vi "Modelo planta H2_V3.vi"() -> ()   [LabVIEW 2024]
uses:
  <vilib>/Modbus/master/Create Master Instance (TCP).vi
  <vilib>/Modbus/master/Modbus Master.lvclass
  <vilib>/OPCUA/NI OPC UA Client.lvlib
  SALICRU_MODBUS.lvlib
  S7-1200_OPCUA.lvlib
panel:
  out "EV6":bool caption="Not initialized"
  out "EV5":bool caption="Not initialized"
  out "EV4":bool caption="Not initialized"
  out "EV3":bool caption="Idle"
  out "EV2":bool caption="Not initialized"
  out "EV1":bool caption="Stand By"
  out "x-y 4":u32
  out "x-y 3":u32
  in  "Restart INV SALICRU com":bool
  in  "Restart SAI com":bool
  out "x-y 2":u32
  in  "stop":bool
  out "x-y":u32
  in  "Tab Control":enum32{"Vista General", "Producción", "Energía"}(tab)
  out "E2.14 2":bool caption="Not initialized"
  out "E1.1":bool caption="Maintenance mode"
  out "E2.2":bool caption="Not initialized"
  out "E2.3":bool caption="Not initialized"
  out "E1.2":bool caption="Maintenance mode"
  out "E1.3":bool caption="Idle"
  out "Prod electrolizadores (display) 4":dbl format="%#.4g"
  out "Prod electrolizadores (display) 3":dbl format="%#.4g"
  out "Prod electrolizadores (display) 2":dbl format="%#.4g"
  out "Potenica Solar (Display) 2":dbl format="%#.2f"
  out "masa total G Kg 2":dbl format="%#.3f"
  out "P alta 2":dbl format="%.1f"
  out "P baja 2":dbl format="%.1f"
  out "masa total P Kg  2":dbl format="%#.3f"
  in  "SAI":bool caption="Line"
  out "Potenica Solar (Display) 3":dbl format="%#.2f"
  out "Comunicacion SAI":bool
  out "E2.1":bool caption="Not initialized"
  out "E2.2":bool caption="Not initialized"
  out "E1.2 2":bool caption="Idle"
  out "E1.1,2":bool caption="Maintenance mode"
  out "E2.1 3":bool caption="Not initialized"
  out "E1.2":bool caption="Maintenance mode"
  out "Producció d'hidrogen":dbl(graph)
  out "Energia solar no utilitzada":dbl(graph)
  out "Pressió tanc baixa":dynamicdata(graph)
  out "Potenica Solar (Display)":dbl format="%#.2f"
  out "Producción FC":dbl format="%#_2g"
  out "Prod electrolizadores (display)":dbl format="%#.4g"
  out "P baja":dbl format="%.1f"
  out "masa total G Kg":dbl format="%#.0f"
  out "Potència inversor solar":dynamicdata(graph)
  out "Watimetro ARPA":dbl format="%#.1f"
  out "masa total P Kg":dbl format="%#.1f"
  out "Compresor":bool
  out "P alta":dbl format="%.1f"
  out "Tèrmic\nExtractors":bool
  out "Relé Seguretat":bool
  out "Sobretensions":bool
  out "Baliza verde":bool
  out "Baliza amarilla":bool
  out "Baliza roja":bool
  out "H2 generado Total":dbl format="%#.1f"
  out "Producción Solar toral":dbl format="%#.1f"
  out "Energía acum H2 verde":dbl format="%#.1f"
  out "H2 consumido en el lab":dbl=182.6 format="%#.1f"
  out "Energía solar diaría":dbl format="%#.1f"
  out "H2 generado dia":dbl format="%#.1f"
  out "Comunicacion Inversor SALICRU":bool
  out "Tank":dbl(slide) scale=0.0..10.0
  out "P tanq alta (barg)":dbl(graph)
  in  "Energía acum H2 verde inicio":dbl=527.0
  in  "Producción Solar total inicio":dbl=3421.0
  in  "H2 generado inicio":dbl=202.8
  out "g H2 consumidos por la FC":dbl
  out "g comprimidos":dbl
  in  "Caudal compresor":dbl
  out "P tanq baja (barg)":dbl(graph)
  in  "Presión ini Tanq baba":dbl=28.0
  in  "Presión ini Tanq alta":dbl=220.0
  out "Energía Solar no usada (kWh)":dbl(graph)
  out "H2 acumulado diario (g)":dbl(graph)
  out "Producción instalan (g/s)":dbl(graph)
  out "Electroli ON":dbl(graph)
  out "Potencia Consumo electroli instan. (kW)":dbl(graph)
  out "Producción diaria (g)":dbl
  out "Producción instalan (g/s)":dbl
  out "Electroli ON":dbl
  out "Potencia Solar Instanta (kW)":dbl(graph)
  # "EV1"
  # "EV4"
  # "ESTADO ELECTROVÁLVULAS"
  # "EV5"
  # "EV2"
  # "EV3"
  # "EV6"
  # "g"
  # "bar"
  # "bar"
  # "kg"
  # "kWh"
  # "kWh"
  # "Ambiente"
  # "Temperatura"
  # "ºC"
  # "Humedad"
  # "%"
  # "ESTADO ELY"
  # "E1.1"
  # "E2.1"
  # "E1.2"
  # "E2.2"
  # "E2.3"
  # "E1.3"
  # "Modo:"
  # "RESUMEN DE LA PRODUCCIÓN"
  # "SAI PLANTA"
  # "Electrolizadores"
  # "Producción\nElectrolizadores:"
  # "g/s"
  # "Inversor solar:"
  # "Energía solar:"
  # "kW"
  # "Tanque Alta"
  # "Presión:"
  # "barg"
  # "Kg"
  # "Capacidad:"
  # "Tanque Baja"
  # "Presión:"
  # "barg"
  # "Kg"
  # "Capacidad:"
  # "SAI:"
  # "Potencia (%):"
  # "%"
  # "Seguretat"
  # "H2 baixa pressió"
  # "H2 alta pressió"
  # "barg"
  # "Tanc baixa pressió"
  # "Tanc alta pressió"
  # "Compressor"
  # "barg"
  # "Solar"
  # "Fuel Cell"
  # "kW"
  # "kW"
  # "Kg"
  # "Kg"
  # "Electrolizadores"
  # "g/s"
  # "Xarxa electrica"
  # "-"
  # "+"
  # "kW de xarxa"
  # "Producció total d'hidrogen"
  # "Producció d'hidrogen diària"
  # "g"
  # "kg"
  # "Producció total d'energia solar"
  # "Energia solar produïda diària"
  # "kWh"
  # "kWh"
  # "Energia acumulada per H2 verd"
  # "Consum de H2 Lab diari"
  # "g"
  # "kWh"
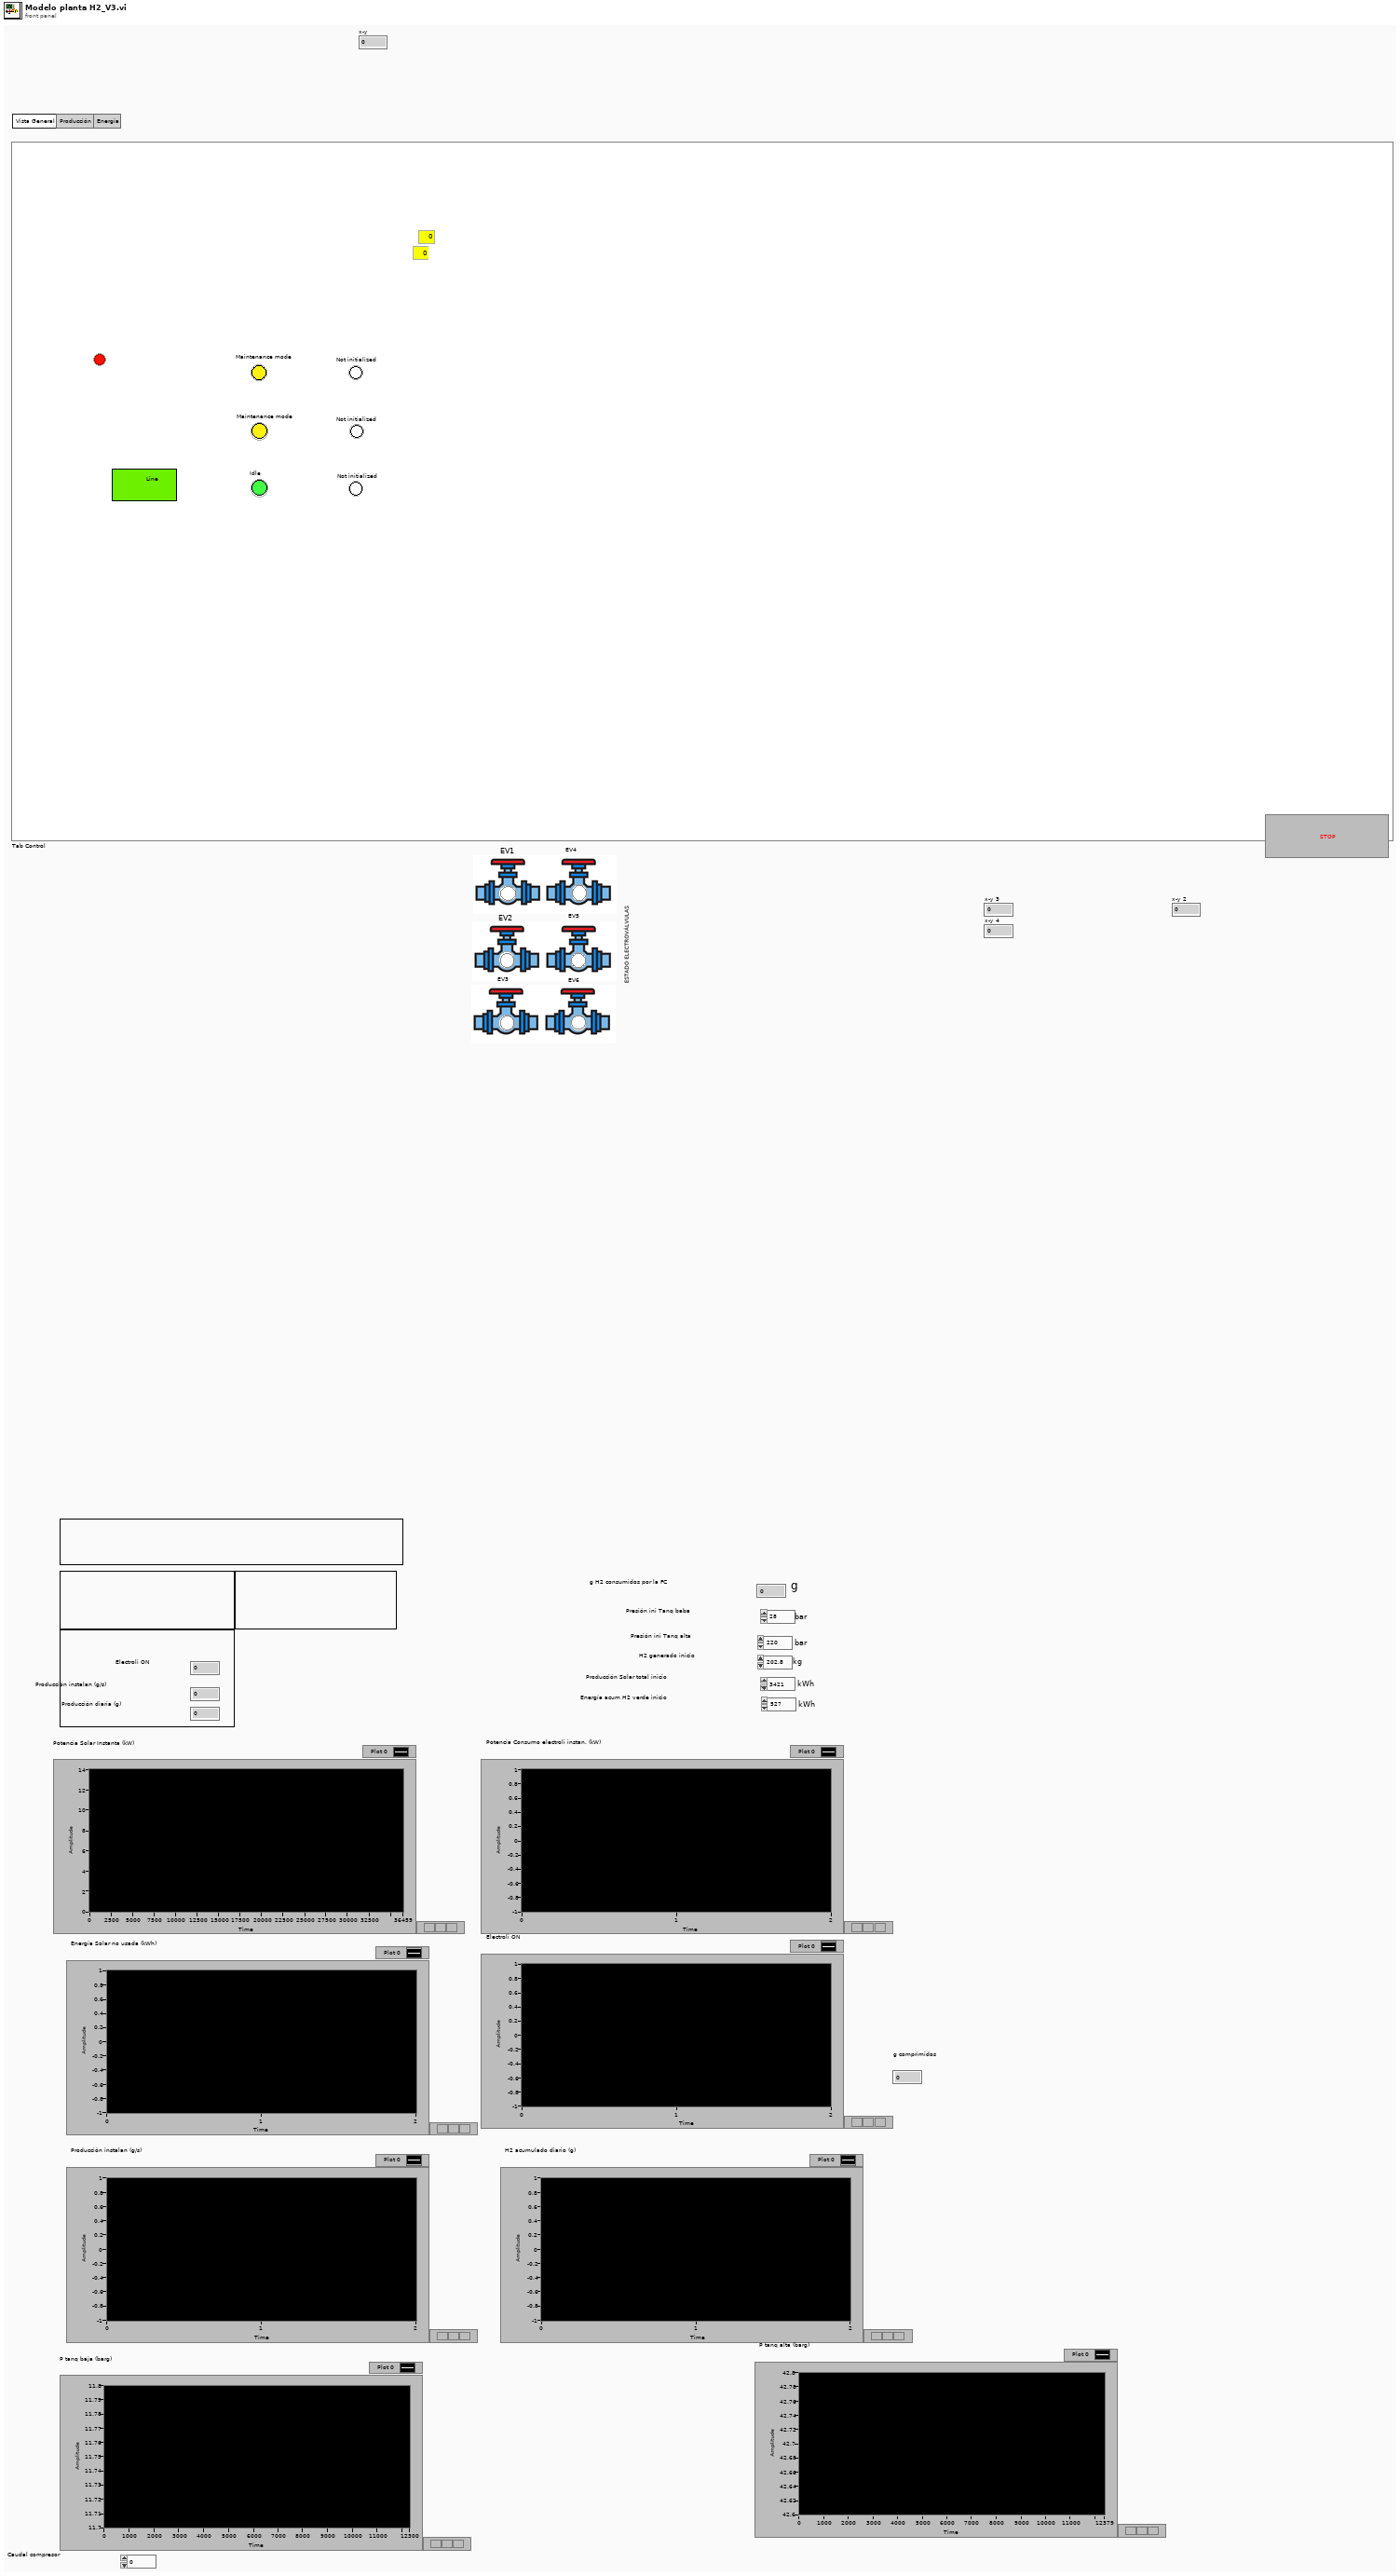
[diagram p1: front panel]
types:
  T1 = cluster{"message mode":enum16{"None", "Sign", "Sign and Encrypt"}, "security":enum16{"Basic256", "Basic128Rsa15"}}
  T2 = typedef "OPC UA Client Refnum.ctl" = refnum<k21>
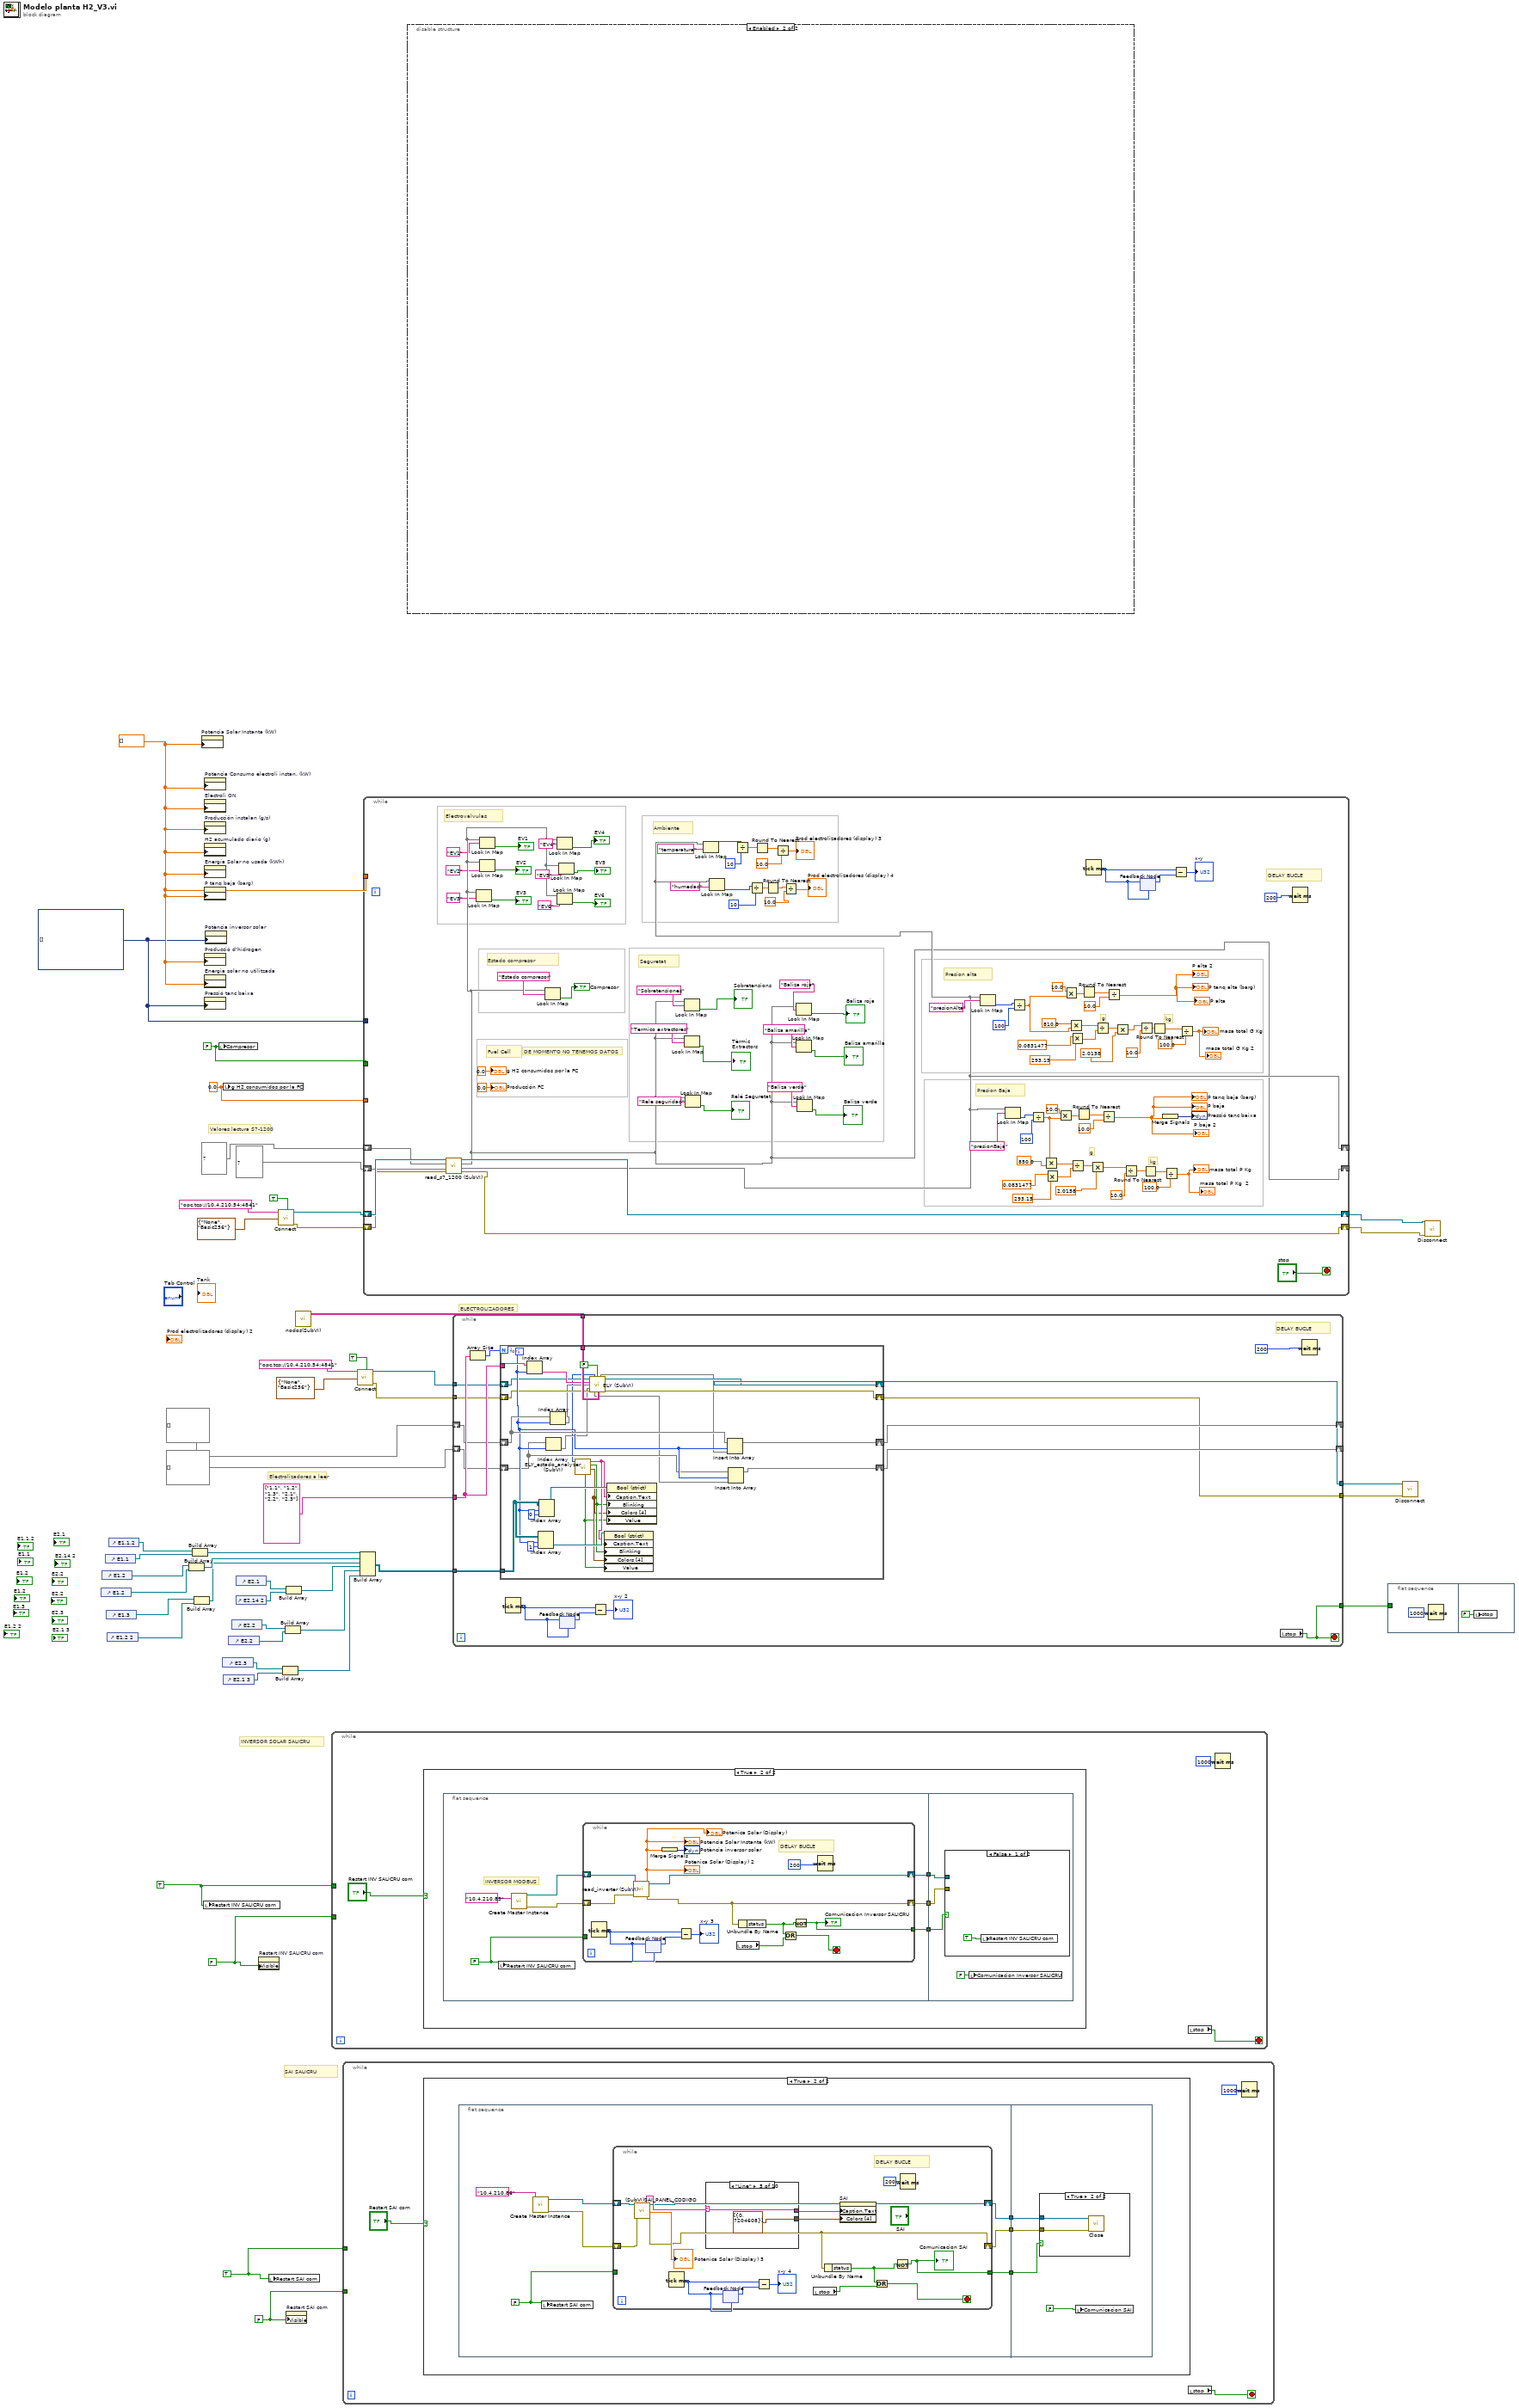
[diagram p0: block diagram]
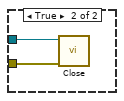
[diagram p3: hidden frame]
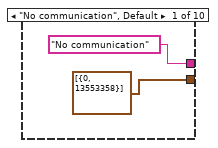
[diagram p5: hidden frame]
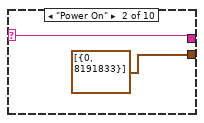
[diagram p6: hidden frame]
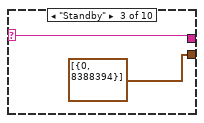
[diagram p7: hidden frame]
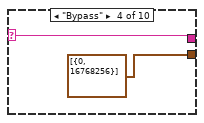
[diagram p8: hidden frame]
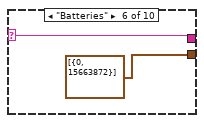
[diagram p9: hidden frame]
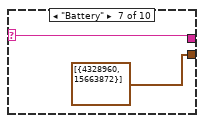
[diagram p10: hidden frame]
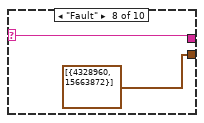
[diagram p11: hidden frame]
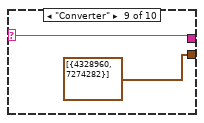
[diagram p12: hidden frame]
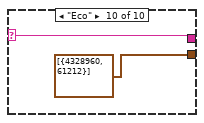
[diagram p13: hidden frame]
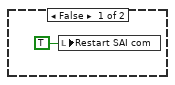
[diagram p14: hidden frame]
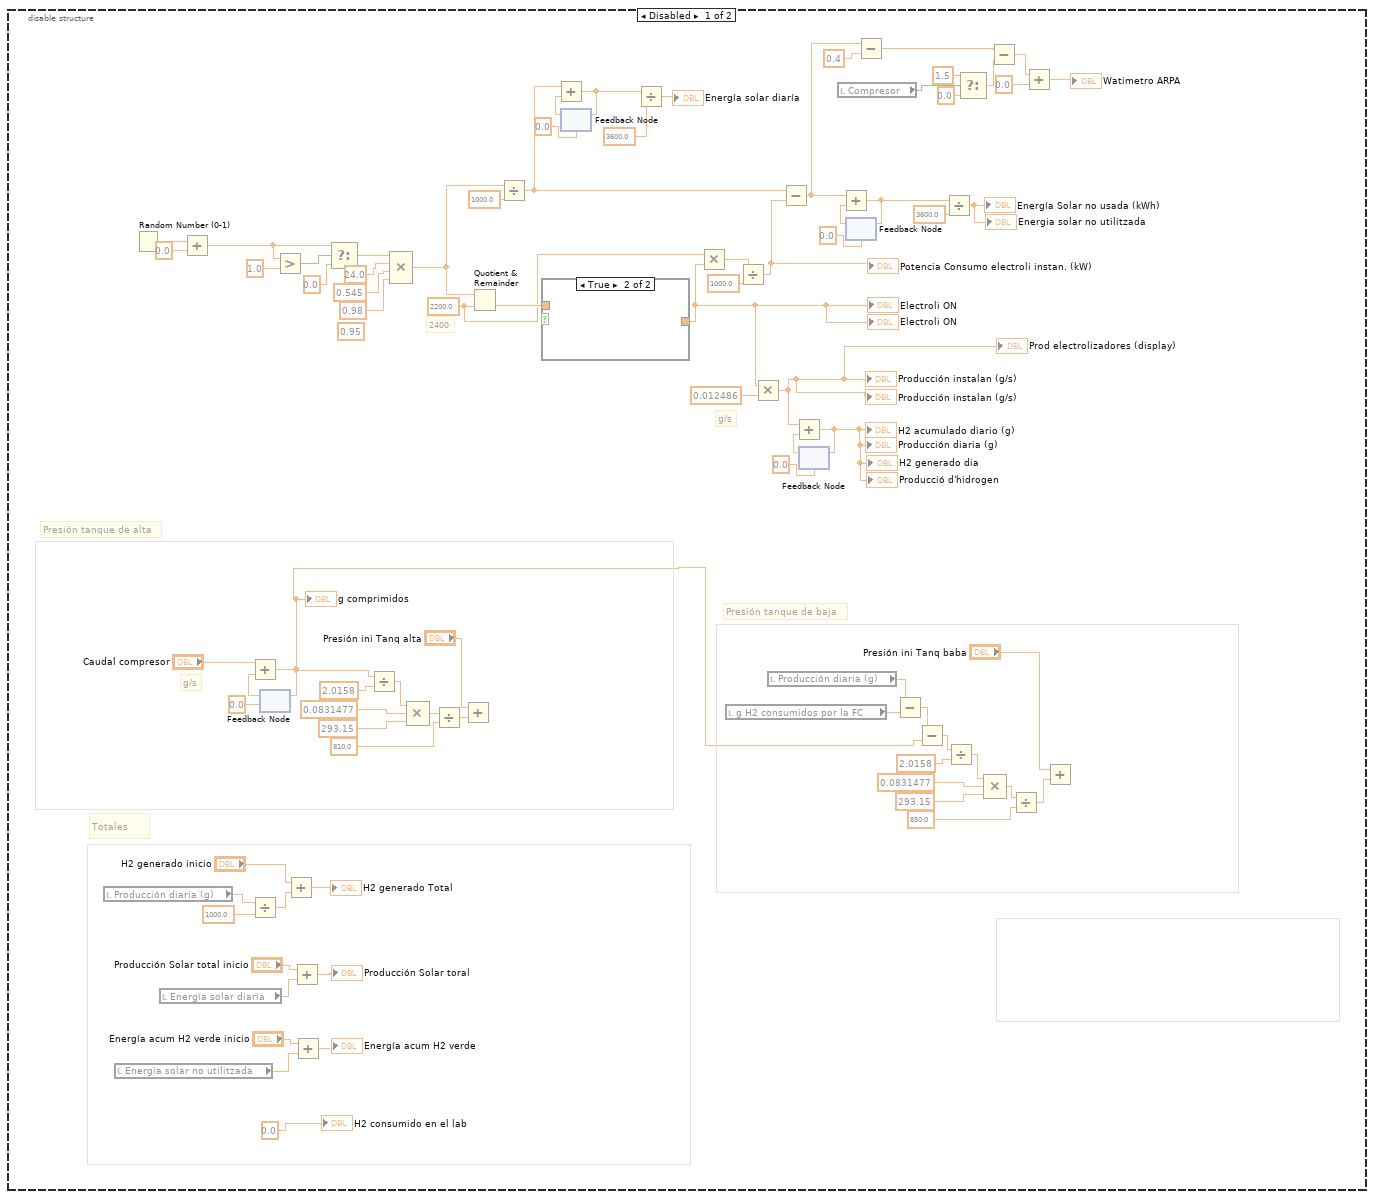
[diagram p15: hidden frame]
diagram:
  w1 = dynamicdata[] [] ("History Data")
  w3 = FALSE ("Visible")
  w4 = FALSE ("Visible")
  w5 = TRUE ("Comunicacion Inversor SALICRU")
  w6 = TRUE ("Restart SAI com")
  w46 = 0.0 ("g H2 consumidos por la FC")
  w47 = FALSE ("Compresor")
  w48 = dbl[] [] ("History Data")
  # "INVERSOR SOLAR SALICRU"
  # "SAI SALICRU"
  # "ELECTROLIZADORES"
  # "Valores lectura S7-1200"
  # "Electrolizadores a leer"
  n1 = control-ref of="E1.2"() -> (w28:refnum<vi>)
  n2 = control-ref of="E1.2"() -> (w27:refnum<vi>)
  n3 = control-ref of="E1.1"() -> (w25:refnum<vi>)
  n4 = control-ref of="E1.3"() -> (w23:refnum<vi>)
  n5 = control-ref of="E1.2 2"() -> (w22:refnum<vi>)
  n6 = control-ref of="E1.1,2"() -> (w24:refnum<vi>)
  n7 = Build Array(w27, w28) -> (w29:refnum<vi>[])
  n8 = Build Array(w24, w25) -> (w26:refnum<vi>[])
  n9 = Build Array(w23, w22) -> (w21:refnum<vi>[])
  n10 = property on="Potencia Solar Instanta (kW)" class="WFChart (strict)"("History Data"=w48) -> ()  [unwired: 2 in, 2 out]
  n11 = local write "Restart INV SALICRU com"(w5) -> ()
  n12 = property on="Potencia Consumo electroli instan. (kW)" class="WFChart (strict)"("History Data"=w48) -> ()  [unwired: 2 in, 2 out]
  n13 = property on="Electroli ON" class="WFChart (strict)"("History Data"=w48) -> ()  [unwired: 2 in, 2 out]
  n14 = property on="Producción instalan (g/s)" class="WFChart (strict)"("History Data"=w48) -> ()  [unwired: 2 in, 2 out]
  n15 = property on="H2 acumulado diario (g)" class="WFChart (strict)"("History Data"=w48) -> ()  [unwired: 2 in, 2 out]
  n16 = property on="Energía Solar no usada (kWh)" class="WFChart (strict)"("History Data"=w48) -> ()  [unwired: 2 in, 2 out]
  n17 = property on="P tanq baja (barg)" class="WFChart (strict)"("History Data"=w48) -> ()  [unwired: 2 in, 2 out]
  n18 = property on="Producció d'hidrogen" class="WFChart (strict)"("History Data"=w48) -> ()  [unwired: 2 in, 2 out]
  n19 = property on="Energia solar no utilitzada" class="WFChart (strict)"("History Data"=w48) -> ()  [unwired: 2 in, 2 out]
  n20 = property on="Pressió tanc baixa" class="WFChart (strict)"("History Data"=w1) -> ()  [unwired: 2 in, 2 out]
  n21 = property on="Potència inversor solar" class="WFChart (strict)"("History Data"=w1) -> ()  [unwired: 2 in, 2 out]
  n22 = local write "Compresor"(w47) -> ()
  n23 = control-ref of="E2.3"() -> (w14:refnum<vi>)
  n24 = local write "g H2 consumidos por la FC"(w46) -> ()
  n25 = control-ref of="E2.1 3"() -> (w13:refnum<vi>)
  n26 = control-ref of="E2.2"() -> (w16:refnum<vi>)
  n27 = control-ref of="E2.2"() -> (w17:refnum<vi>)
  n28 = control-ref of="E2.1"() -> (w20:refnum<vi>)
  n29 = control-ref of="E2.14 2"() -> (w19:refnum<vi>)
  n30 = property on="Restart INV SALICRU com" class="Bool (strict)"("Visible"=w4) -> ()  [unwired: 2 in, 2 out]
  n31 = local write "Restart SAI com"(w6) -> ()
  n32 = call <vilib>:"Connect.vi"("trust any server (F)"=TRUE, "security policy"=T1 {"message mode"=enum."None", "security"=enum."Basic256"}, "server endpoint URL"="opc.tcp://10.4.210.54:4841") -> ("error out"=w38:errorcluster, "OPC UA client refnum out"=w39:T2)  [unwired: 6 in, 1 out]
  n33 = Build Array(w14, w13) -> (w12:refnum<vi>[])
  n34 = Build Array(w17, w16) -> (w15:refnum<vi>[])
  n35 = Build Array(w20, w19) -> (w18:refnum<vi>[])
  n36 = property on="Restart SAI com" class="Bool (strict)"("Visible"=w3) -> ()  [unwired: 2 in, 2 out]
  n37 = call "nodos(SubVI).vi"() -> ("Array"=w7:string[][])  [unwired: 11 in]
  n38 = while {
    tunnel: w5 -> [_]
    tunnel: w4 -> [_]
    stop <- w50 stop-if-true
    n39 = case shown="True" "Restart INV SALICRU com" {
      frame False {
      }
      frame True {
        n40 = flat-sequence {
          tunnel: [w60] -> w54
          tunnel: [w57] -> w53
          tunnel: [w56] -> w52
          tunnel: w54 -> [w79]
          tunnel: w53 -> [w78]
          tunnel: w52 -> [w77]
          frame #0 {
            w55 = FALSE ("Restart INV SALICRU com")
            # "INVERSOR MODBUS"
            n41 = local write "Restart INV SALICRU com"(w55) -> ()
            n42 = call-poly <vilib>:"Create Master Instance.vi"("address"="10.4.210.85") -> ("error out"=w58:errorcluster, "TCP master instance"=w59:refnum<class "Modbus Master.lvclass">)  [unwired: 9 in]
            n43 = while {
              shift-right: [w64] -> w57
              shift-left: w59 -> [w75]
              shift-right: [w72] -> w60
              shift-left: w58 -> [w74]
              tunnel: [w68] -> w56
              tunnel: w55 -> [_]
              stop <- w70 stop-if-true
              # "DELAY BUCLE"
              n44 = Tick Count (ms)() -> (millisecond timer value=w67:u32)
              n45 = call "read_inverter (SubVI).vi"("error in (no error)"=w74, "Modbus Master in"=w75) -> ("error out"=w72:errorcluster, "Inverter kW"=w62:dbl, "Modbus Master out"=w64:refnum<class "Modbus Master.lvclass">)  [unwired: 7 in]
              "Potencia Solar Instanta (kW)" <- w62
              "Potenica Solar (Display)" <- w62
              "Potenica Solar (Display) 2" <- w62
              n46 = feedback #1(w67) -> (w66:u32)
              n47 = feedback-in #1(w67) -> ()
              n48 = Merge Signals(w62) -> (→"Potència inversor solar":dynamicdata)
              n49 = Subtract(x=w67, y=w66) -> (x-y=→"x-y 3":u32)
              n50 = local read "stop"() -> (w71:bool)
              n51 = Unbundle By Name(w72) -> ("status"=w69:bool)
              n52 = Or(x=w69, y=w71) -> (x .or. y?=w70:bool)
              n53 = Not(x=w69) -> (.not. x?=w68:bool)
              "Comunicacion Inversor SALICRU" <- w68
              n54 = Wait (ms)(milliseconds to wait=u32 200) -> ()  [unwired: 1 out]
            }
          }
          frame #1 {
            n55 = case shown="False" w77 {
              tunnel: w79 -> [_ w82]
              tunnel: w78 -> [_ w81]
              frame False {
                n56 = local write "Restart INV SALICRU com"(TRUE ("Restart INV SALICRU com")) -> ()
              }
              frame True {
                n57 = call-dynamic "Close.vi"("error in (no error)"=w82, "Modbus master in"=w81) -> ()  [unwired: 9 in, 1 out]
              }
            }
            n58 = local write "Comunicacion Inversor SALICRU"(FALSE ("Comunicacion Inversor SALICRU")) -> ()
          }
        }
      }
    }
    n59 = local read "stop"() -> (w50:bool)
    n60 = Wait (ms)(milliseconds to wait=u32 1000) -> ()  [unwired: 1 out]
  }
  n61 = while {
    tunnel: w6 -> [_]
    tunnel: w3 -> [_]
    stop <- w84 stop-if-true
    n62 = case shown="True" "Restart SAI com" {
      frame False {
      }
      frame True {
        n63 = flat-sequence {
          tunnel: [w92] -> w88
          tunnel: [w91] -> w87
          tunnel: [w90] -> w86
          tunnel: w88 -> [w135]
          tunnel: w87 -> [w134]
          tunnel: w86 -> [w133]
          frame #0 {
            w89 = FALSE ("Restart SAI com")
            n64 = call-poly <vilib>:"Create Master Instance.vi"("address"="10.4.210.86") -> ("error out"=w93:errorcluster, "TCP master instance"=w94:refnum<class "Modbus Master.lvclass">)  [unwired: 9 in]
            n65 = local write "Restart SAI com"(w89) -> ()
            n66 = while {
              shift-right: [w105] -> w91
              shift-left: w94 -> [w107]
              shift-right: [w103] -> w92
              shift-left: w93 -> [w106]
              tunnel: [w99] -> w90
              tunnel: w89 -> [_]
              stop <- w101 stop-if-true
              # "DELAY BUCLE"
              n67 = call "(SubVI)SAI_PANEL_CODIGO.vi"("Modbus Master in"=w107, "error in (no error)"=w106) -> ("Work mode"=w108:string, "Modbus Master out"=w105:refnum<class "Modbus Master.lvclass">, "Porcentaje P"=→"Potenica Solar (Display) 3":dbl, "error out"=w103:errorcluster)  [unwired: 4 in, 10 out]
              n68 = Tick Count (ms)() -> (millisecond timer value=w98:u32)
              n69 = case shown="\"Line\"" w108 {
                selector: w108 -> [_ w115 w117 w119 w121 w123 w125 w127 w129 w131]
                tunnel: ["No communication" w115 w117 w119 w121 w123 w125 w127 w129 w131] -> w109
                tunnel: [cluster{u32, u32}[] [{0, 13553358}] ("Colors [4]") cluster{u32, u32}[] [{0, 8191833}] ("Colors [4]") cluster{u32, u32}[] [{0, 8388394}] ("Colors [4]") cluster{u32, u32}[] [{0, 16768256}] ("Colors [4]") cluster{u32, u32}[] [{0, 7204608}] ("Colors [4]") cluster{u32, u32}[] [{0, 15663872}] ("Colors [4]") cluster{u32, u32}[] [{4328960, 15663872}] ("Colors [4]") cluster{u32, u32}[] [{4328960, 15663872}] ("Colors [4]") cluster{u32, u32}[] [{4328960, 7274282}] ("Colors [4]") cluster{u32, u32}[] [{4328960, 61212}] ("Colors [4]")] -> w110
                frame "No communication", Default {
                }
                frame "Power On" {
                }
                frame "Standby" {
                }
                frame "Bypass" {
                }
                frame "Line" {
                }
                frame "Batteries" {
                }
                frame "Battery" {
                }
                frame "Fault" {
                }
                frame "Converter" {
                }
                frame "Eco" {
                }
              }
              n70 = feedback #2(w98) -> (w97:u32)
              n71 = feedback-in #2(w98) -> ()
              n72 = Subtract(x=w98, y=w97) -> (x-y=→"x-y 4":u32)
              n73 = local read "stop"() -> (w102:bool)
              n74 = Unbundle By Name(w103) -> ("status"=w100:bool)
              n75 = property on="SAI" class="Bool"("Caption.Text"=w109, "Colors [4]"=w110) -> ()  [unwired: 2 in, 2 out]
              n76 = Or(x=w100, y=w102) -> (x .or. y?=w101:bool)
              n77 = Not(x=w100) -> (.not. x?=w99:bool)
              "Comunicacion SAI" <- w99
              n78 = Wait (ms)(milliseconds to wait=u32 200) -> ()  [unwired: 1 out]
            }
          }
          frame #1 {
            n79 = case shown="True" w133 {
              tunnel: w135 -> [_ w138]
              tunnel: w134 -> [_ w137]
              frame False {
                n80 = local write "Restart SAI com"(TRUE ("Restart SAI com")) -> ()
              }
              frame True {
                n81 = call-dynamic "Close.vi"("error in (no error)"=w138, "Modbus master in"=w137) -> ()  [unwired: 9 in, 1 out]
              }
            }
            n82 = local write "Comunicacion SAI"(FALSE) -> ()
          }
        }
      }
    }
    n83 = local read "stop"() -> (w84:bool)
    n84 = Wait (ms)(milliseconds to wait=u32 1000) -> ()  [unwired: 1 out]
  }
  n85 = call <vilib>:"Connect.vi"("trust any server (F)"=TRUE, "security policy"=T1 {"message mode"=enum."None", "security"=enum."Basic256"}, "server endpoint URL"="opc.tcp://10.4.210.54:4841") -> ("error out"=w33:errorcluster, "OPC UA client refnum out"=w34:T2)  [unwired: 6 in, 1 out]
  n86 = Build Array(w26, w29, w21, w18, w15, w12) -> (w11:refnum<vi>[][])
  n87 = while {
    tunnel: w48 -> [_]
    tunnel: w47 -> [_]
    tunnel: w46 -> [_]
    shift-right: [w193] -> w32
    shift-left: w39 -> [w238]
    shift-right: [w141] -> w31
    shift-left: w38 -> [w237]
    shift-right: [w182] -> _
    shift-left: map{string, bool} {} ("Coils in") -> [w195]
    shift-right: [w190] -> _
    shift-left: map{string, i32} {} ("Values in") -> [w196]
    tunnel: w1 -> [_]
    stop <- "stop" stop-if-true
    # "g"
    # "kg"
    # "kg"
    # "g"
    # "Electrovalvulas"
    # "Ambiente"
    # "DELAY BUCLE"
    # "Seguretat"
    # "Presion Baja"
    # "Presion alta"
    # "DE MOMENTO NO TENEMOS DATOS"
    # "Fuel Cell"
    # "Estado compresor"
    n88 = call "read_s7_1200 (SubVI).vi"("error in (no error)"=w237, "Coils in"=w195, "Values in"=w196, "Refnum in"=w238) -> ("error out"=w141:errorcluster, "VALUES READ"=w190:map{string, i32}, "Coils read"=w182:map{string, bool}, "Refnum out"=w193:T2)  [unwired: 4 in]
    n89 = Look In Map(map=w182, key="EV3") -> (value=→"EV3":bool)  [unwired: 1 in, 1 out]
    n90 = Look In Map(map=w182, key="EV1") -> (value=→"EV1":bool)  [unwired: 1 in, 1 out]
    n91 = Look In Map(map=w182, key="EV2") -> (value=→"EV2":bool)  [unwired: 1 in, 1 out]
    n92 = Look In Map(map=w182, key="Estado compresor") -> (value=→"Compresor":bool)  [unwired: 1 in, 1 out]
    n93 = Look In Map(map=w182, key="EV4") -> (value=→"EV4":bool)  [unwired: 1 in, 1 out]
    n94 = Look In Map(map=w182, key="EV6") -> (value=→"EV6":bool)  [unwired: 1 in, 1 out]
    n95 = Look In Map(map=w182, key="EV5") -> (value=→"EV5":bool)  [unwired: 1 in, 1 out]
    n96 = Look In Map(map=w182, key="Sobretensiones") -> (value=→"Sobretensions":bool)  [unwired: 1 in, 1 out]
    n97 = Look In Map(map=w182, key="Termico extractores") -> (value=→"Tèrmic\nExtractors":bool)  [unwired: 1 in, 1 out]
    n98 = Look In Map(map=w182, key="Rele seguridad") -> (value=→"Relé Seguretat":bool)  [unwired: 1 in, 1 out]
    n99 = Look In Map(map=w190, key="temperatura") -> (value=w189:i32)  [unwired: 1 in, 1 out]
    n100 = Look In Map(map=w190, key="humedad") -> (value=w187:i32)  [unwired: 1 in, 1 out]
    n101 = Divide(x=w189, y=10) -> (x/y=w172:dbl)
    n102 = Divide(x=w187, y=10) -> (x/y=w165:dbl)
    n103 = Round To Nearest(number=w172) -> (nearest integer value=w171:dbl)
    n104 = Round To Nearest(number=w165) -> (nearest integer value=w168:dbl)
    n105 = Divide(x=w171, y=10.0) -> (x/y=→"Prod electrolizadores (display) 3":dbl)
    n106 = Divide(x=w168, y=10.0) -> (x/y=→"Prod electrolizadores (display) 4":dbl)
    n107 = Look In Map(map=w182, key="Baliza roja") -> (value=→"Baliza roja":bool)  [unwired: 1 in, 1 out]
    n108 = Look In Map(map=w182, key="Baliza amarilla") -> (value=→"Baliza amarilla":bool)  [unwired: 1 in, 1 out]
    n109 = Look In Map(map=w182, key="Baliza verde") -> (value=→"Baliza verde":bool)  [unwired: 1 in, 1 out]
    n110 = Look In Map(map=w190, key="presionAlta") -> (value=w218:i32)  [unwired: 1 in, 1 out]
    n111 = Look In Map(map=w190, key="presionBaja") -> (value=w216:i32)  [unwired: 1 in, 1 out]
    n112 = Divide(x=w218, y=100) -> (x/y=w144:dbl)
    n113 = Divide(x=w216, y=100) -> (x/y=w152:dbl)
    n114 = Multiply(x=w152, y=850.0) -> (x*y=w207:dbl)
    n115 = Multiply(x=0.0831477 ("y"), y=293.15) -> (x*y=w205:dbl)
    n116 = Multiply(x=10.0, y=w152) -> (x*y=w148:dbl)
    n117 = Multiply(x=10.0, y=w144) -> (x*y=w145:dbl)
    n118 = Multiply(x=810.0 ("y"), y=w144) -> (x*y=w210:dbl)
    n119 = Multiply(x=0.0831477 ("y"), y=293.15) -> (x*y=w213:dbl)
    n120 = Divide(x=w207, y=w205) -> (x/y=w204:dbl)
    n121 = Round To Nearest(number=w148) -> (nearest integer value=w150:dbl)
    n122 = Round To Nearest(number=w145) -> (nearest integer value=w146:dbl)
    n123 = Tick Count (ms)() -> (millisecond timer value=w200:u32)
    n124 = Multiply(x=w204, y=2.0158) -> (x*y=w154:dbl)
    n125 = Divide(x=w210, y=w213) -> (x/y=w214:dbl)
    n126 = Divide(x=w150, y=10.0) -> (x/y=w140:dbl)
    "P tanq baja (barg)" <- w140
    "P baja" <- w140
    "P baja 2" <- w140
    n127 = Divide(x=w146, y=10.0) -> (x/y=→"P tanq alta (barg)" →"P alta" →"P alta 2":dbl)
    n128 = Multiply(x=w214, y=2.0158) -> (x*y=w160:dbl)
    n129 = Divide(x=w154, y=10.0) -> (x/y=w158:dbl)
    n130 = Divide(x=w160, y=10.0) -> (x/y=w164:dbl)
    n131 = feedback-in #3(w200) -> ()
    n132 = feedback #3(w200) -> (w199:u32)
    n133 = Round To Nearest(number=w158) -> (nearest integer value=w157:dbl)
    n134 = Round To Nearest(number=w164) -> (nearest integer value=w163:dbl)
    n135 = Merge Signals(w140) -> (→"Pressió tanc baixa":dynamicdata)
    n136 = Divide(x=w157, y=100.0) -> (x/y=→"masa total P Kg" →"masa total P Kg  2":dbl)
    n137 = Subtract(x=w200, y=w199) -> (x-y=→"x-y":u32)
    n138 = Divide(x=w163, y=100.0) -> (x/y=→"masa total G Kg" →"masa total G Kg 2":dbl)
    n139 = Wait (ms)(milliseconds to wait=u32 200) -> ()  [unwired: 1 out]
    "Producción FC" <- 0.0 ("Producción FC")
    "g H2 consumidos por la FC" <- 0.0 ("g H2 consumidos por la FC")
  }
  n140 = disable-structure shown="Enabled" {
    frame Disabled {
      (unwired) 0.95 ("f")
      w255 = 2200.0 ("y")
      # "Totales"
      # "g/s"
      # "2400"
      # "g/s"
      # "Presión tanque de alta"
      # "Presión tanque de baja"
      n141 = local read "Producción diaria (g)"() -> (w250:dbl)
      n142 = local read "Energia solar no utilitzada"() -> (w241:dbl)
      n143 = Random Number (0-1)() -> (number: 0 to 1=w266:dbl)
      n144 = local read "Energía solar diaría"() -> (w245:dbl)
      n145 = Add(x=w266, y=0.0) -> (x+y=w267:dbl)
      n146 = Divide(x=w250, y=1000.0) -> (x/y=w249:dbl)
      n147 = feedback #4(0.0) -> (w313:dbl)
      n148 = Add(x="Caudal compresor", y=w313) -> (x+y=w309:dbl)
      "g comprimidos" <- w309
      n149 = feedback-in #4(w309) -> ()
      n150 = Greater?(x=w267, y=1.0) -> (0:w268:bool)
      n151 = Add(x="H2 generado inicio", y=w249) -> (x+y=→"H2 generado Total":dbl)
      n152 = Add(x="Producción Solar total inicio", y=w245) -> (x+y=→"Producción Solar toral":dbl)
      n153 = Add(x="Energía acum H2 verde inicio", y=w241) -> (x+y=→"Energía acum H2 verde":dbl)
      n154 = Select(t=w267, s=w268, f=0.0) -> (s? t:f=w269:dbl)
      n155 = Divide(x=w309, y=2.0158) -> (x/y=w307:dbl)
      n156 = Compound Arithmetic op=MULTIPLY(w269, 24.0 ("f"), 0.545 ("f"), 0.98 ("f")) -> (w277:dbl)
      n157 = Compound Arithmetic op=MULTIPLY(w307, 0.0831477 ("y"), 293.15 ("y")) -> (w317:dbl)
      n158 = Divide(x=w317, y=810.0) -> (x/y=w316:dbl)
      n159 = Add(x="Presión ini Tanq alta", y=w316) -> (x+y=w311:dbl)
      n160 = Quotient & Remainder(x=w277, y=w255) -> (floor(x/y)=w276:dbl)  [unwired: 1 out]
      n161 = Divide(x=w277, y=1000.0) -> (x/y=w292:dbl)
      n162 = case shown="True" {
        selector: _ -> [_ _]
        tunnel: w276 -> [w321 _]
        tunnel: [w321 _] -> w282
        frame False {
        }
        frame True {
        }
      }
      "Electroli ON" <- w282
      "Electroli ON" <- w282
      n163 = feedback #5(0.0) -> (w291:dbl)
      n164 = Add(x=w292, y=w291) -> (x+y=w290:dbl)
      n165 = feedback-in #5(w290) -> ()
      n166 = Divide(x=w290, y=3600.0) -> (x/y=→"Energía solar diaría":dbl)
      n167 = Multiply(x=w255, y=w282) -> (x*y=w278:dbl)
      n168 = local read "g H2 consumidos por la FC"() -> (w296:dbl)
      n169 = Divide(x=w278, y=1000.0) -> (x/y=w279:dbl)
      "Potencia Consumo electroli instan. (kW)" <- w279
      n170 = Multiply(x=w282, y=0.012486) -> (x*y=w280:dbl)
      "Producción instalan (g/s)" <- w280
      "Producción instalan (g/s)" <- w280
      "Prod electrolizadores (display)" <- w280
      n171 = local read "Producción diaria (g)"() -> (w298:dbl)
      n172 = Subtract(x=w292, y=w279) -> (x-y=w283:dbl)
      n173 = feedback #6(0.0) -> (w273:dbl)
      n174 = Add(x=w280, y=w273) -> (x+y=w294:dbl)
      "Producción diaria (g)" <- w294
      "H2 acumulado diario (g)" <- w294
      "Producció d'hidrogen" <- w294
      "H2 generado dia" <- w294
      n175 = feedback-in #6(w294) -> ()
      n176 = local read "Compresor"() -> (w284:bool)
      n177 = feedback #7(0.0) -> (w274:dbl)
      n178 = Add(x=w283, y=w274) -> (x+y=w275:dbl)
      n179 = feedback-in #7(w275) -> ()
      n180 = Subtract(x=w283, y=0.4) -> (x-y=w286:dbl)
      n181 = Subtract(x=w298, y=w296) -> (x-y=w297:dbl)
      n182 = Subtract(x=w297, y=w309) -> (x-y=w301:dbl)
      n183 = Divide(x=w275, y=3600.0) -> (x/y=→"Energía Solar no usada (kWh)" →"Energia solar no utilitzada":dbl)
      n184 = Divide(x=w301, y=2.0158) -> (x/y=w306:dbl)
      n185 = Select(t=1.5, s=w284, f=0.0 ("t")) -> (s? t:f=w285:dbl)
      n186 = Compound Arithmetic op=MULTIPLY(w306, 0.0831477 ("y"), 293.15 ("y")) -> (w304:dbl)
      n187 = Subtract(x=w286, y=w285) -> (x-y=w287:dbl)
      n188 = Divide(x=w304, y=850.0) -> (x/y=w300:dbl)
      n189 = Add(x=w287, y=0.0) -> (x+y=→"Watimetro ARPA":dbl)
      n190 = Add(x="Presión ini Tanq baba", y=w300) -> (x+y=w295:dbl)
      "H2 consumido en el lab" <- 0.0 ("H2 consumido en el lab")
    }
    frame Enabled {
    }
  }
  n191 = while {
    tunnel: string[] ["1.1", "1.2", "1.3", "2.1", "2.2", "2.3"] -> [w337]
    tunnel: w34 -> [w336]
    tunnel: w33 -> [w335]
    tunnel: [w334] -> w30
    tunnel: w11 -> [w330]
    tunnel: [w323] -> w10
    shift-right: [w326] -> _
    shift-left: map{string, dbl}[] [] -> [w328]
    shift-right: [w325] -> _
    shift-left: map{string, dbl}[] [] -> [w327]
    tunnel: w7 -> [w324]
    tunnel: [w322] -> w2
    stop <- w322 stop-if-true
    # "DELAY BUCLE"
    n192 = Array Size(array=w337) -> (size(s)=w338:i32)
    n193 = for {
      N: w338 -> [_]
      shift-right: [w344] -> w334
      shift-left: w336 -> [w348]
      shift-right: [w343] -> w323
      shift-left: w335 -> [w347]
      tunnel: w337 -> [w365]
      tunnel: w330 -> [w364]
      shift-right: [w354] -> w326
      shift-left: w328 -> [w355]
      shift-right: [w351] -> w325
      shift-left: w327 -> [w352]
      tunnel: w324 -> [w350]
      i -> [w353]
      n194 = Index Array(array=w365, index=w353) -> (element=w349:string)
      n195 = Index Array(array=w364, index (row)=w353, index (col)=1 ("disabled index (col)")) -> (element=w360:refnum<vi>)
      n196 = Index Array(array=w364, index (row)=w353, index (col)=0 ("disabled index (col)")) -> (element=w361:refnum<vi>)
      n197 = Index Array(array=w352, index=w353) -> (element=w345:map{string, dbl})
      n198 = Index Array(array=w355, index=w353) -> (element=w346:map{string, dbl})
      n199 = call "ELY (SubVI).vi"("Refnum in"=w348, "Leer mas¿?"=FALSE, "Electrolizador"=w349, "Produccion in"=w346, "Medidas in"=w345, "error in (no error)"=w347, "Nodos"=w350) -> ("Estado"=w340:u16, "Produccion"=w342:map{string, dbl}, "Refnum out"=w344:T2, "Medidas"=w341:map{string, dbl}, "error out"=w343:errorcluster)  [unwired: 1 in, 3 out]
      n200 = call "ELY_estado_analyzer (SubVI).vi"("Numeric"=w340) -> ("Colors [4]"=w357:cluster{u32, u32}[], "Boolean 2"=w358:bool, "Caption.Text"=w359:string, "Boolean"=w356:bool)  [unwired: 7 in]
      n201 = property class="Bool (strict)"(reference=w360, "Caption.Text"=w359, "Blinking"=w358, "Colors [4]"=w357, "Value"=w356) -> ()  [unwired: 1 in, 2 out]
      n202 = property class="Bool (strict)"(reference=w361, "Caption.Text"=w359, "Blinking"=w358, "Colors [4]"=w357, "Value"=w356) -> ()  [unwired: 1 in, 2 out]
      n203 = Insert Into Array(array=w355, index=w353, new element=w342) -> (w354:map{string, dbl}[])
      n204 = Insert Into Array(array=w352, index=w353, new element=w341) -> (w351:map{string, dbl}[])
    }
    n205 = Tick Count (ms)() -> (millisecond timer value=w333:u32)
    n206 = feedback #8(w333) -> (w332:u32)
    n207 = feedback-in #8(w333) -> ()
    n208 = Subtract(x=w333, y=w332) -> (x-y=→"x-y 2":u32)
    n209 = local read "stop"() -> (w322:bool)
    n210 = Wait (ms)(milliseconds to wait=u32 200) -> ()  [unwired: 1 out]
  }
  n211 = flat-sequence {
    tunnel: w2 -> [_]
    frame #0 {
      n212 = Wait (ms)(milliseconds to wait=u32 1000) -> ()  [unwired: 1 out]
    }
    frame #1 {
      n213 = local write "stop"(FALSE ("stop")) -> ()
    }
  }
  n214 = call <vilib>:"Disconnect.vi"("error in (no error)"=w10, "OPC UA client refnum in"=w30) -> ()  [unwired: 9 in, 1 out]
  n215 = call <vilib>:"Disconnect.vi"("error in (no error)"=w31, "OPC UA client refnum in"=w32) -> ()  [unwired: 9 in, 1 out]
